vi "Controle_Manip_Main_GUI_WorkingBackup_211222.vi"() -> ()   [LabVIEW 2019] (continued)
                      n490 = property class="Page"(reference=w548, "PageVis"=TRUE ("Page Visible")) -> ()  [unwired: 1 in, 2 out]
                      n491 = property class="Page"(reference=w552, "PageVis"=TRUE ("Page Visible")) -> ()  [unwired: 1 in, 2 out]
                    }
                    frame False {
                      n492 = property on="Experimental parameters tab" class="TabCtl (strict)"() -> ("Pages"=w557:refnum<vi>[])  [unwired: 2 in, 2 out]
                      n493 = property on="Experiment Graph Controls" class="TabCtl (strict)" props=["Value", "Pages"]() -> ("Pages"=w558:refnum<vi>[])  [unwired: 2 in, 3 out]
                      n494 = Index Array(array=w557, index=3) -> (element=w556:refnum<vi>)
                      n495 = Index Array(array=w558, index=3) -> (element=w560:refnum<vi>)
                      n496 = property class="Page"(reference=w556, "PageVis"=FALSE ("Page Visible")) -> ()  [unwired: 1 in, 2 out]
                      n497 = property class="Page"(reference=w560, "PageVis"=FALSE ("Page Visible")) -> ()  [unwired: 1 in, 2 out]
                    }
                  }
                }
                frame True {
                  n498 = stacked-sequence {
                    frame #0 {
                      w577 = TRUE
                      w576 = FALSE
                      n499 = property on="Experiment Graph Controls" class="TabCtl (strict)"("Value"=T25."Contrast" ("Experiment Graph Controls")) -> ("Pages"=w572:refnum<vi>[])  [unwired: 2 in, 2 out]
                      n500 = property on="Experimental parameters tab" class="TabCtl (strict)"("Value"=T19."Translation" ("Experimental parameters tab")) -> ("Pages"=w571:refnum<vi>[])  [unwired: 2 in, 2 out]
                      n501 = local read "Log file"() -> (w567:string)
                      n502 = Index Array(array=w572, index=3) -> (element=w574:refnum<vi>)
                      n503 = Index Array(array=w571, index=3) -> (element=w568:refnum<vi>)
                      n504 = property class="Page"(reference=w574, "PageVis"=TRUE ("Page Visible")) -> ()  [unwired: 1 in, 2 out]
                      n505 = property on="Stop Contrast" class="Bool (strict)"("Visible"=w576) -> ()  [unwired: 2 in, 2 out]
                      n506 = property on="Pause Contrast" class="Bool (strict)"("Visible"=w576) -> ()  [unwired: 2 in, 2 out]
                      n507 = property class="Page"(reference=w568, "PageVis"=TRUE ("Page Visible")) -> ()  [unwired: 1 in, 2 out]
                      n508 = call "Write2LogFile.vi"("Add to log file"="Initialise communication with PZC", "Log file before"=w567, "Checkbox"=FALSE) -> ("Log file after"=w566:string)
                      n509 = local write "Log file"(w566) -> ()
                      n510 = local read "Scan Contrast Ctrls"() -> (w579:refnum<vi>[])
                      n511 = property on="Save Contrast" class="Bool (strict)"("Visible"=w577) -> ()  [unwired: 2 in, 2 out]
                      n512 = property on="Acquire Contrast" class="Bool (strict)"("Visible"=w577) -> ()  [unwired: 2 in, 2 out]
                      n513 = call "Enable&Disable_Controls.vi"("Enum"=enum16{"Enabled", "Disabled", "Disabled&Grayed"}."Enabled", "References"=w579) -> ()  [unwired: 1 in]
                    }
                    frame #1 {
                      # "RS232/10"
                      n514 = local read "PZC200 COM Port"() -> (w581:dbl)
                      n515 = call "Create Instrument Channel.vi"("XON/XOFF Handshaking(F)"=TRUE, "Baud Rate (38400)"=u32 19200, "COM Port (1)"=w581, "(T) - GPIB, F - RS232"=FALSE) -> ("Instrument Channel out"=w585:string)  [unwired: 5 in, 2 out]
                      n516 = call "SendCommand.vi"("Command"="1TS?", "Instrument Channel"=w585) -> ("Instrument Channel out"=w586:string)  [unwired: 8 in, 1 out]
                      n517 = call "ReadCommand.vi"("Disable MAV check (F)"=TRUE, "Instrument Channel"=w586) -> ("Response"=w587:string, "Instrument Channel out"=w580:string)  [unwired: 7 in, 1 out]
                      "Response" <- w587
                      n518 = String Length(string=w587) -> (length=w594:i32)
                      n519 = Subtract(x=w594, y=1) -> (x-y=w592:i32)
                      n520 = local write "PZC200 Instrument Channel"(w580) -> ()
                      n521 = String Subset(string=w587, offset (0)=w592) -> (substring=w591:string)  [unwired: 1 in]
                      n522 = case shown="\"@\", Default" w591 {
                        tunnel: [FALSE TRUE TRUE] -> w590
                        frame "@", Default {
                        }
                        frame "Q" {
                        }
                        frame "P" {
                        }
                      }
                      n523 = local write "LinTFine Motor On?"(w590) -> ()
                      n524 = call "PZCGetPos.vi"("Instrument Channel"=w580) -> ("Position"=w588:i32)  [unwired: 1 in, 2 out]
                      n525 = local write "PZC Position Readout (usteps)"(w588) -> ()
                    }
                  }
                }
              }
            }
            frame #15 {
              # "Advance progress bar"
              n526 = local write "Scan Main Progess Bar"(u8 85 ("Scan Main Progess Bar")) -> ()
            }
            frame #16 {
              # "Attocube ANC350 with 2 ANPx51 and 1 ANPz51"
              n527 = case shown="True" "Attocubes On?" {
                tunnel: [FALSE ("Page Visible") TRUE] -> w600
                frame False {
                }
                frame True {
                  n528 = stacked-sequence {
                    frame #0 {
                      n529 = control-ref of="Experimental parameters tab"() -> (w610:refnum<vi>)
                      n530 = property class="TabCtl (strict)"(reference=w610, "Value"=T19."Microscope objective") -> ()  [unwired: 1 in, 2 out]
                      n531 = local read "Log file"() -> (w614:string)
                      n532 = control-ref of="Tab Objective Sample"() -> (w612:refnum<vi>)
                      n533 = call "Write2LogFile.vi"("Add to log file"="Initialise communication with ANC350", "Log file before"=w614, "Checkbox"=FALSE) -> ("Log file after"=w615:string)
                      n534 = local write "Log file"(w615) -> ()
                      n535 = property class="TabCtl (strict)"(reference=w612, "Value"=T22."Sample piezo stack") -> ()  [unwired: 1 in, 2 out]
                      "ourDLL" <- path "C:/Users/manip/Documents/Controle_Manip_2020/subVIs/Attocubes/anc350v4.dll"
                    }
                    frame #1 {
                      w620 = u32 1 items=["None", "USB", "TCP", "All"] ("Interface types")
                      n536 = local read "ourDLL"() -> (w617:path)
                      n537 = call "ANC350v4_Discover.vi"("Path to *.DLL"=w617, "Interface types"=w620) -> ("ANC350v4 found"=w619:u32, "error ANC350v4_discover"=w618:errorcluster)  [unwired: 12 in]
                      n538 = case shown="1" w619 {
                        tunnel: w618 -> [_ w622]
                        tunnel: w617 -> [_ w621]
                        frame 0, Default {
                        }
                        frame 1 {
                          n539 = stacked-sequence {
                            seq-local: [w624 _] -> [_ w655]
                            seq-local: [w623 _] -> [_ w654]
                            tunnel: w622 -> [w641 _]
                            tunnel: w621 -> [w630 w653]
                            frame #0 {
                              w625 = u8 0 items=["1", "2", "3"] ("axis")
                              w628 = u8 2 items=["1", "2", "3"] ("axis")
                              w629 = u8 1 items=["1", "2", "3"] ("axis")
                              n540 = call "ANC350v4sub_Connect.vi"("Path to *.DLL"=w630, "deviceNumber"=0, "error in"=w641) -> ("ANC350v4_Handle_Out"=w637:u64, "error ANC350v4_Dis/Connect"=w640:errorcluster)  [unwired: 11 in]
                              n541 = call "ANC350v4_GetDeviceInfo.vi"("Path to *.DLL"=w630, "deviceNumber"=u32 0, "error in"=w640) -> ("connected"=→"ANC connected":bool, "Error_ANC350v4_getDeviceInfo"=w636:errorcluster)  [unwired: 5 in, 6 out]
                              n542 = call "ANC350v4_GetPosition.vi"("deviceHandle"=w637, "Path to *.DLL"=w630, "axis"=w625, "error in"=w636) -> ("deviceHandle"=w634:u64, "Position [µm | m°]"=w635:dbl, "error ANC350v4_getPosition"=w633:errorcluster)  [unwired: 8 in, 1 out]
                              n543 = local write "Att Pos Y"(w635) -> ()
                              n544 = call "ANC350v4_GetPosition.vi"("deviceHandle"=w634, "Path to *.DLL"=w630, "axis"=w629, "error in"=w633) -> ("deviceHandle"=w632:u64, "Position [µm | m°]"=w626:dbl, "error ANC350v4_getPosition"=w631:errorcluster)  [unwired: 8 in, 1 out]
                              n545 = local write "Att Pos X"(w626) -> ()
                              n546 = call "ANC350v4_GetPosition.vi"("deviceHandle"=w632, "Path to *.DLL"=w630, "axis"=w628, "error in"=w631) -> ("deviceHandle"=w624:u64, "Position [µm | m°]"=w627:dbl, "error ANC350v4_getPosition"=w623:errorcluster)  [unwired: 8 in, 1 out]
                              n547 = local write "Att Pos Z"(w627) -> ()
                            }
                            frame #1 {
                              w643 = u8 2 items=["1", "2", "3"] ("axis")
                              w644 = u8 1 items=["1", "2", "3"] ("axis")
                              w645 = u8 0 items=["1", "2", "3"] ("axis")
                              w652 = 0.1 ("TargetRange [µm | m°]")
                              # "Define Target resolution in um"
                              n548 = call "ANC350v4_SetTargetRange.vi"("deviceHandle"=w655, "Path to *.DLL"=w653, "axis"=w645, "TargetRange [µm | m°]"=w652, "error in"=w654) -> ("deviceHandle"=w651:u64, "error ANC350v4_setTargetRange"=w649:errorcluster)  [unwired: 8 in, 1 out]
                              n549 = call "ANC350v4_SetTargetRange.vi"("deviceHandle"=w651, "Path to *.DLL"=w653, "axis"=w644, "TargetRange [µm | m°]"=w652, "error in"=w649) -> ("deviceHandle"=w650:u64, "error ANC350v4_setTargetRange"=w648:errorcluster)  [unwired: 8 in, 1 out]
                              n550 = call "ANC350v4_SetTargetRange.vi"("deviceHandle"=w650, "Path to *.DLL"=w653, "axis"=w643, "TargetRange [µm | m°]"=w652, "error in"=w648) -> ("deviceHandle"=→"Att DeviceHandle":u64, "error ANC350v4_setTargetRange"=→"Att Error":errorcluster)  [unwired: 8 in, 1 out]
                            }
                          }
                        }
                      }
                    }
                  }
                }
              }
              n551 = control-ref of="Tab Objective Sample"() -> (w602:refnum<vi>)
              n552 = property class="TabCtl (strict)"(reference=w602) -> ("Pages"=w603:refnum<vi>[])  [unwired: 1 in, 2 out]
              n553 = Index Array(array=w603, index=1) -> (element=w604:refnum<vi>)
              n554 = property class="Page"(reference=w604, "PageVis"=w600) -> ()  [unwired: 1 in, 2 out]
            }
            frame #17 {
              # "Montana Cryostation s50"
              n555 = case shown="True" "Cryostation On?" {
                frame False {
                }
                frame True {
                  w671 = 10.0 ("y")
                  n556 = call "CryoConnect.vi"() -> ("connection ID"=w661:refnum<k5>)
                  "Cryostation ID" <- w661
                  n557 = local read "Log file"() -> (w660:string)
                  n558 = call "Write2LogFile.vi"("Add to log file"="Initialise communication with Cryostation", "Log file before"=w660, "Checkbox"=FALSE) -> ("Log file after"=w659:string)
                  n559 = local write "Log file"(w659) -> ()
                  n560 = call "GetCryoInfo.vi"("connection ID"=w661) -> ("User Stability"=w666:dbl, "User Temp"=w665:dbl, "connection ID out"=w667:refnum<k5>, "Sample Stability"=w664:dbl, "Sample Temp"=w668:dbl, "Platform Stability"=w663:dbl, "Platform Temp"=w662:dbl)  [unwired: 4 in]
                  n561 = local write "Cryo Platform Temp"(w662) -> ()
                  n562 = Multiply(x=w668, y=w671) -> (x*y=w669:dbl)
                  n563 = local write "Cryo Sample Stability"(w664) -> ()
                  n564 = local write "Cryostation ID"(w667) -> ()
                  n565 = local write "Cryo User Stability"(w666) -> ()
                  n566 = local write "Cryo Sample Temp"(w668) -> ()
                  n567 = local write "Cryo Platform Stability"(w663) -> ()
                  n568 = local write "Cryo User Temp"(w665) -> ()
                  n569 = Round To Nearest(number=w669) -> (nearest integer value=w670:dbl)
                  n570 = Divide(x=w670, y=w671) -> (x/y=w672:dbl)
                  n571 = local write "Temperature (K)"(w672) -> ()
                }
              }
            }
            frame #18 {
              # "PicoHarp"
              n572 = case shown="True" "PicoHarp On?" {
                frame False {
                  n573 = local write "Connected"(FALSE) -> ()
                }
                frame True {
                  n574 = local read "Log file"() -> (w684:string)
                  n575 = property on="Experiment Graph Controls" class="TabCtl (strict)"("Value"=T25."APDs" ("Experiment Graph Controls")) -> ("Pages"=w679:refnum<vi>[])  [unwired: 2 in, 2 out]
                  n576 = call "Write2LogFile.vi"("Add to log file"="Initialise communication with PicoHarp", "Log file before"=w684, "Checkbox"=FALSE) -> ("Log file after"=w683:string)
                  n577 = call "PH_Init.vi"() -> ("PH_Init_Data"=→"PH_Init_Data":T11)
                  n578 = local write "Log file"(w683) -> ()
                  n579 = Index Array(array=w679, index=4) -> (element=w680:refnum<vi>)
                  n580 = property class="Page"(reference=w680, "PageVis"=TRUE ("Page Visible")) -> ()  [unwired: 1 in, 2 out]
                  n581 = local write "Connected"(TRUE) -> ()
                }
              }
            }
            frame #19 {
              # "Final activation message"
              n582 = local read "Log file"() -> (w690:string)
              n583 = property on="Experiment Graph Controls" class="TabCtl (strict)"("Value"=T25."Settings" ("Experiment Graph Controls")) -> ()  [unwired: 2 in, 2 out]
              n584 = call "Write2LogFile.vi"("Add to log file"="All devices activated !", "Log file before"=w690, "Checkbox"=FALSE) -> ("Log file after"=w691:string)
              n585 = local write "Log file"(w691) -> ()
              n586 = local write "Scan Main Progess Bar"(u8 100 ("Scan Main Progess Bar")) -> ()
            }
            frame #20 {
              # "Autosave Init"
              n587 = local read "Auto< ?"() -> (w692:bool)
              n588 = case shown="True" w692 {
                frame False {
                  w693 = TRUE ("Visible")
                  n589 = property on="Save Spectrum N" class="Bool (strict)"("Visible"=w693) -> ()  [unwired: 2 in, 2 out]
                  n590 = property on="Save XY Map" class="Bool (strict)"("Visible"=w693) -> ()  [unwired: 2 in, 2 out]
                  n591 = property on="Save Spectrum" class="Bool (strict)"("Visible"=w693) -> ()  [unwired: 2 in, 2 out]
                  n592 = property on="Save PLE" class="Bool (strict)"("Visible"=w693) -> ()  [unwired: 2 in, 2 out]
                  n593 = property on="Save fPow" class="Bool (strict)"("Visible"=w693) -> ()  [unwired: 2 in, 2 out]
                  n594 = property on="Save Custom Diode Spectrum" class="Bool (strict)"("Visible"=w693) -> ()  [unwired: 2 in, 2 out]
                  n595 = property on="Save Michelson" class="Bool (strict)"("Visible"=w693) -> ()  [unwired: 2 in, 2 out]
                  n596 = property on="Save Polarisation" class="Bool (strict)"("Visible"=w693) -> ()  [unwired: 2 in, 2 out]
                  n597 = property on="Save Contrast" class="Bool (strict)"("Visible"=w693) -> ()  [unwired: 2 in, 2 out]
                }
                frame True {
                  w694 = FALSE ("Visible")
                  n598 = property on="Save Spectrum N" class="Bool (strict)"("Visible"=w694) -> ()  [unwired: 2 in, 2 out]
                  n599 = property on="Save XY Map" class="Bool (strict)"("Visible"=w694) -> ()  [unwired: 2 in, 2 out]
                  n600 = property on="Save Spectrum" class="Bool (strict)"("Visible"=w694) -> ()  [unwired: 2 in, 2 out]
                  n601 = property on="Save PLE" class="Bool (strict)"("Visible"=w694) -> ()  [unwired: 2 in, 2 out]
                  n602 = property on="Save fPow" class="Bool (strict)"("Visible"=w694) -> ()  [unwired: 2 in, 2 out]
                  n603 = property on="Save Polarisation" class="Bool (strict)"("Visible"=w694) -> ()  [unwired: 2 in, 2 out]
                  n604 = property on="Save Michelson" class="Bool (strict)"("Visible"=w694) -> ()  [unwired: 2 in, 2 out]
                  n605 = property on="Save Contrast" class="Bool (strict)"("Visible"=w694) -> ()  [unwired: 2 in, 2 out]
                  n606 = property on="Save Custom Diode Spectrum" class="Bool (strict)"("Visible"=w694) -> ()  [unwired: 2 in, 2 out]
                }
              }
            }
          }
        }
      }
    }
    frame #2 {
      # "Main Program"
      n607 = while {
        stop <- w846 stop-if-true
        # "Main loop with unique event structure handling nearly all events (that needn't happen at the same time)"
        n608 = event shown="[0] \"Acquire Time Trace\", \"Acquire Polarisation\", \"Acquire XY Map\", \"Acquire Contrast\", \"Acquire Michelson\", \"Acquire Spectrum\", \"Fast Acq\", \"Acquire Custom Diode Spectrum\", \"Acquire fPow\", \"Acquire PLE\": Mouse Down" {
          selector: _ -> [_ _ _ _ _ _ _ _ _ _ _ _ _ _ _ _ _ _ _ _ _ _ _ _ _ _ _ _ _ _ _ _ _ _ _ _ _ _ _ _ _ _ _ _ _ _ _ _ _ _ _ _ _ _]
          dyn-events: _ -> [_ _ _ _ _ _ _ _ _ _ _ _ _ _ _ _ _ _ _ _ _ _ _ _ _ _ _ _ _ _ _ _ _ _ _ _ _ _ _ _ _ _ _ _ _ _ _ _ _ _ _ _ _ _]
          timeout: 500 -> [_ _ _ _ _ _ _ _ _ _ _ _ _ _ _ _ _ _ _ _ _ _ _ _ _ _ _ _ _ _ _ _ _ _ _ _ _ _ _ _ _ _ _ _ _ _ _ _ _ _ _ _ _ _]
          tunnel: [_ _ _ _ _ _ _ _ _ _ _ _ _ _ _ _ _ _ _ _ _ _ _ _ _ _ _ _ _ _ _ _ _ _ _ _ _ _ _ _ _ _ _ _ _ _ _ _ w4459 _ _ _ _ _] -> w846
          event "Acquire Time Trace", "Acquire Polarisation", "Acquire XY Map", "Acquire Contrast", "Acquire Michelson", "Acquire Spectrum", "Fast Acq", "Acquire Custom Diode Spectrum", "Acquire fPow", "Acquire PLE": Mouse Down {
            # "FAILLE\naucune protection \nde trigger si ESP et \nPicoHarp mais pas LF"
            # "Launch an acquisition or an experiment"
            n609 = event-data() -> ("CtlRef"=w852:refnum<vi>)  [unwired: 1 in, 7 out]
            n610 = local read "LightField On?"() -> (w849:bool)
            n611 = local read "PicoHarp On?"() -> (w850:bool)
            n612 = local read "ESP 300 On?"() -> (w851:bool)
            n613 = And(x=w851, y=w850) -> (x .and. y?=w848:bool)
            n614 = Or(x=w849, y=w848) -> (x .or. y?=w847:bool)
            n615 = stacked-sequence {
              tunnel: w852 -> [w854 w2750]
              tunnel: w847 -> [w853 _]
              frame #0 {
                # "Actual measurements"
                n616 = case shown="True" w853 {
                  tunnel: w854 -> [_ w859]
                  frame False {
                    n617 = local read "Log file"() -> (w858:string)
                    n618 = call "Write2LogFile.vi"("Add to log file"="LightField not activated; cannot acquire", "Log file before"=w858, "Checkbox"=FALSE) -> ("Log file after"=w857:string)
                    n619 = local write "Log file"(w857) -> ()
                  }
                  frame True {
                    n620 = property class="Bool"(reference=w859) -> ("Label.Text"=w860:string)  [unwired: 1 in, 2 out]
                    n621 = case shown="\"Acquire XY Map\"" w860 {
                      frame "Acquire Spectrum", Default {
                        n622 = stacked-sequence {
                          frame #0 {
                            # "background"
                            n623 = local read "Background taken?"() -> (w861:bool)
                            n624 = case shown="False" w861 {
                              frame False {
                                n625 = stacked-sequence {
                                tunnel: [_ _ w907] -> w862
                                frame #0 {
                                n626 = property on="CCD 1D Spectrum Main" class="XYGraph (strict)"("YScale.Offset"=0.0 ("Y Scale.Offset and Multiplier:Offset")) -> ()  [unwired: 2 in, 2 out]
                                }
                                frame #1 {
                                # "make sure shutter is closed"
                                n627 = local read "KCube Shutter On?"() -> (w893:bool)
                                n628 = control-ref of="Shutter Ctrls"() -> (w897:refnum<vi>)
                                n629 = property class="Ring (strict)"(reference=w897) -> ("Value"=w896:u16)  [unwired: 1 in, 2 out]
                                n630 = control-ref of="KCube Shutter Device Reference"() -> (w898:refnum<vi>)
                                n631 = Equal?(x=w896, y=u16 0) -> (x = y?=w894:bool)
                                n632 = case shown="False" w894 {
                                tunnel: w898 -> [w901 _]
                                tunnel: w897 -> [w900 _]
                                tunnel: w893 -> [w899 _]
                                frame False {
                                n633 = call "Shutter.vi"("KCube Shutter Device Reference 2"=w901, "Shutter Ctrls 2"=w900, "Shutter on?"=w899) -> ()
                                }
                                frame True {
                                }
                                }
                                }
                                frame #2 {
                                # "acquire"
                                n634 = local read "LightField Automation error out"() -> (w905:errorcluster)
                                n635 = local read "LightField Automation out"() -> (w906:refnum<class "LightField Automation.lvclass">)
                                n636 = local read "Accumulations"() -> (w902:dbl)
                                n637 = call "LFA_Capture.vi"("error in (no error)"=w905, "Frames"=w902, "LightField Automation in"=w906) -> ("error out"=w904:errorcluster, "Data"=w907:T26, "LightField Automation out"=w903:refnum<class "LightField Automation.lvclass">)  [unwired: 6 in]
                                n638 = local write "LightField Automation error out"(w904) -> ()
                                n639 = local write "LightField Automation out"(w903) -> ()
                                }
                                }
                                n640 = local read "Acq Mode"() -> (w863:T3)
                                n641 = case shown="\"Spectrum\", Default" w863 {
                                selector: w863 -> [w864 w882]
                                tunnel: w862 -> [w865 w883]
                                frame "Spectrum", Default {
                                n642 = stacked-sequence {
                                tunnel: w865 -> [_ w876 _ _]
                                tunnel: w864 -> [_ w874 _ _]
                                frame #0 {
                                n643 = property on="CCD 2D Image Main" class="IntGraph (strict)"("Visible"=FALSE) -> ()  [unwired: 2 in, 2 out]
                                n644 = property on="CCD 1D Spectrum Main" class="XYGraph (strict)"("Visible"=TRUE) -> ()  [unwired: 2 in, 2 out]
                                }
                                frame #1 {
                                n645 = local read "Wavelength calibration"() -> (w873:dbl[])
                                n646 = local read "CCD ROI"() -> (w869:T20)
                                n647 = Divide(x=1239.842, y=w873) -> (x/y=w871:dbl[])
                                n648 = call "PrepareData4Graph.vi"("Wavelength nm"=w871, "DataLF"=w876, "CCD ROI"=w869, "AcqMode"=w874, "Data type"=T30."Spectre") -> ("Spectrum"=w875:cluster{"Array 2":dbl[], "Array":dbl[]}, "PLInt out"=w868:dbl[])  [unwired: 2 in, 2 out]
                                n649 = local write "CCD 1D Spectrum Main"(w875) -> ()
                                n650 = local write "BackgroundSpec"(w868) -> ()
                                }
                                frame #2 {
                                n651 = local read "BackgroundSpec"() -> (w877:dbl[])
                                n652 = call-poly <vilib>:"Mean.vi"("X"=w877) -> ("mean"=w879:dbl)  [unwired: 1 out]
                                n653 = Negate(x=w879) -> (-x=w878:dbl)
                                n654 = property on="CCD 1D Spectrum Main" class="XYGraph (strict)"("YScale.Offset"=w878) -> ()  [unwired: 2 in, 2 out]
                                }
                                frame #3 {
                                n655 = local write "Background taken?"(TRUE ("Background taken?")) -> ()
                                n656 = property on="Background substract" class="Enum (strict)"("Value"=enum16{"None", "Shutter"}."None" ("Background substract")) -> ()  [unwired: 2 in, 2 out]
                                }
                                }
                                }
                                frame "Image" {
                                n657 = stacked-sequence {
                                tunnel: w883 -> [_ w891]
                                tunnel: w882 -> [_ w889]
                                frame #0 {
                                n658 = property on="CCD 1D Spectrum Main" class="XYGraph (strict)"("Visible"=FALSE) -> ()  [unwired: 2 in, 2 out]
                                n659 = property on="CCD 2D Image Main" class="IntGraph (strict)"("Visible"=TRUE) -> ()  [unwired: 2 in, 2 out]
                                }
                                frame #1 {
                                n660 = local read "Wavelength calibration"() -> (w890:dbl[])
                                n661 = local read "CCD ROI"() -> (w886:T20)
                                n662 = call "PrepareData4Graph.vi"("Wavelength nm"=w890, "DataLF"=w891, "CCD ROI"=w886, "AcqMode"=w889, "Data type"=T30."Spectre") -> ("Intensity Graph"=w888:dbl[][])  [unwired: 2 in, 3 out]
                                n663 = local write "CCD 2D Image Main"(w888) -> ()
                                }
                                }
                                }
                                }
                              }
                              frame True {
                              }
                            }
                          }
                          frame #1 {
                            # "measurement"
                            n664 = stacked-sequence {
                              frame #0 {
                                # "open shutter if closed"
                                n665 = control-ref of="KCube Shutter Device Reference"() -> (w910:refnum<vi>)
                                n666 = control-ref of="Shutter Ctrls"() -> (w909:refnum<vi>)
                                n667 = property class="Ring (strict)"(reference=w909) -> ("Value"=w911:u16)  [unwired: 1 in, 2 out]
                                n668 = local read "KCube Shutter On?"() -> (w914:bool)
                                n669 = Equal?(x=w911, y=u16 0) -> (x = y?=w913:bool)
                                n670 = property on="Experiment Graph Controls" class="TabCtl (strict)"("Value"=T25."Spectrum" ("Experiment Graph Controls")) -> ()  [unwired: 2 in, 2 out]
                                n671 = case shown="True" w913 {
                                tunnel: w910 -> [_ w917]
                                tunnel: w909 -> [_ w916]
                                tunnel: w914 -> [_ w915]
                                frame False {
                                }
                                frame True {
                                n672 = call "Shutter.vi"("KCube Shutter Device Reference 2"=w917, "Shutter Ctrls 2"=w916, "Shutter on?"=w915) -> ()
                                }
                                }
                              }
                              frame #1 {
                                # "set CCD ROI and acquire"
                                n673 = local read "LightField Automation error out"() -> (w926:errorcluster)
                                n674 = local read "LightField Automation out"() -> (w918:refnum<class "LightField Automation.lvclass">)
                                n675 = local read "CCD ROI"() -> (w925:T20)
                                n676 = local read "Accumulations"() -> (w922:dbl)
                                n677 = call "Adv_SetROI.vi"("error in (no error)"=w926, "ROI"=w925, "LightField Automation in"=w918) -> ("error out"=w923:errorcluster, "LightField Automation out"=w924:refnum<class "LightField Automation.lvclass">)  [unwired: 7 in]
                                n678 = call "LFA_Capture.vi"("error in (no error)"=w923, "Frames"=w922, "LightField Automation in"=w924) -> ("error out"=w921:errorcluster, "Data"=w920:T26, "LightField Automation out"=w919:refnum<class "LightField Automation.lvclass">)  [unwired: 6 in]
                                n679 = local write "LightField Automation out"(w919) -> ()
                                n680 = local write "LightField Automation error out"(w921) -> ()
                                n681 = local write "Data"(w920) -> ()
                              }
                              frame #2 {
                                # "close shutter"
                                n682 = local read "KCube Shutter On?"() -> (w929:bool)
                                n683 = control-ref of="KCube Shutter Device Reference"() -> (w928:refnum<vi>)
                                n684 = control-ref of="Shutter Ctrls"() -> (w927:refnum<vi>)
                                n685 = call "Shutter.vi"("KCube Shutter Device Reference 2"=w928, "Shutter Ctrls 2"=w927, "Shutter on?"=w929) -> ()
                              }
                              frame #3 {
                                # "Show data accordingly"
                                n686 = local read "Data"() -> (w930:T26)
                                n687 = local read "Acq Mode"() -> (w931:T3)
                                n688 = case shown="\"Spectrum\", Default" w931 {
                                selector: w931 -> [w932 w951]
                                tunnel: w930 -> [w933 w952]
                                frame "Spectrum", Default {
                                n689 = stacked-sequence {
                                tunnel: w933 -> [_ w949 _]
                                tunnel: w932 -> [_ w948 _]
                                frame #0 {
                                n690 = property on="CCD 1D Spectrum Main" class="XYGraph (strict)"("Visible"=TRUE) -> ()  [unwired: 2 in, 2 out]
                                n691 = property on="CCD 2D Image Main" class="IntGraph (strict)"("Visible"=FALSE) -> ()  [unwired: 2 in, 2 out]
                                }
                                frame #1 {
                                n692 = local read "Wavelength calibration"() -> (w947:dbl[])
                                n693 = local read "CCD ROI"() -> (w943:T20)
                                n694 = local read "BackgroundSpec"() -> (w937:dbl[])
                                n695 = Divide(x=1239.842, y=w947) -> (x/y=w945:dbl[])
                                n696 = call "PrepareData4Graph.vi"("BackgroundSpec"=w937, "Wavelength nm"=w945, "DataLF"=w949, "CCD ROI"=w943, "AcqMode"=w948, "Data type"=T30."Spectre") -> ("Spectrum"=w936:cluster{"Array 2":dbl[], "Array":dbl[]}, "PLInt out"=w941:dbl[])  [unwired: 1 in, 2 out]
                                n697 = control-ref of="Cnts"() -> (w942:refnum<vi>)
                                n698 = local read "Excitation Power (uW)"() -> (w939:dbl)
                                n699 = local write "CCD 1D Spectrum Main"(w936) -> ()
                                n700 = local read "Acq Time (ms)"() -> (w940:dbl)
                                n701 = local read "Display Mode"() -> (w938:u16)
                                n702 = call "2Cnts.vi"("Array Background"=w937, "Pow W"=w939, "AcqTime ms"=w940, "Cnts Ref"=w942, "Display Mode"=w938, "Array"=w941) -> ()  [unwired: 1 out]
                                }
                                frame #2 {
                                n703 = property on="Full scale" class="Bool (strict)"("Val(Sgnl)"=TRUE ("Value (Signaling)")) -> ()  [unwired: 2 in, 2 out]
                                }
                                }
                                }
                                frame "Image" {
                                n704 = stacked-sequence {
                                tunnel: w952 -> [_ w960]
                                tunnel: w951 -> [_ w958]
                                frame #0 {
                                n705 = property on="CCD 1D Spectrum Main" class="XYGraph (strict)"("Visible"=FALSE) -> ()  [unwired: 2 in, 2 out]
                                n706 = property on="CCD 2D Image Main" class="IntGraph (strict)"("Visible"=TRUE) -> ()  [unwired: 2 in, 2 out]
                                }
                                frame #1 {
                                n707 = local read "Wavelength calibration"() -> (w959:dbl[])
                                n708 = local read "CCD ROI"() -> (w955:T20)
                                n709 = call "PrepareData4Graph.vi"("Wavelength nm"=w959, "DataLF"=w960, "CCD ROI"=w955, "AcqMode"=w958, "Data type"=T30."Spectre") -> ("Intensity Graph"=w957:dbl[][])  [unwired: 2 in, 3 out]
                                n710 = local write "CCD 2D Image Main"(w957) -> ()
                                }
                                }
                                }
                                }
                              }
                            }
                          }
                        }
                      }
                      frame "Acquire fPow" {
                        n711 = stacked-sequence {
                          frame #0 {
                            # "background"
                            n712 = local read "Background taken?"() -> (w961:bool)
                            n713 = case shown="False" w961 {
                              frame False {
                                n714 = stacked-sequence {
                                tunnel: [_ _ w1007] -> w962
                                frame #0 {
                                n715 = property on="CCD 1D Spectrum Main" class="XYGraph (strict)"("YScale.Offset"=0.0 ("Y Scale.Offset and Multiplier:Offset")) -> ()  [unwired: 2 in, 2 out]
                                }
                                frame #1 {
                                # "make sure shutter is closed"
                                n716 = local read "KCube Shutter On?"() -> (w993:bool)
                                n717 = control-ref of="Shutter Ctrls"() -> (w997:refnum<vi>)
                                n718 = property class="Ring (strict)"(reference=w997) -> ("Value"=w996:u16)  [unwired: 1 in, 2 out]
                                n719 = control-ref of="KCube Shutter Device Reference"() -> (w998:refnum<vi>)
                                n720 = Equal?(x=w996, y=u16 0) -> (x = y?=w994:bool)
                                n721 = case shown="False" w994 {
                                tunnel: w998 -> [w1001 _]
                                tunnel: w997 -> [w1000 _]
                                tunnel: w993 -> [w999 _]
                                frame False {
                                n722 = call "Shutter.vi"("KCube Shutter Device Reference 2"=w1001, "Shutter Ctrls 2"=w1000, "Shutter on?"=w999) -> ()
                                }
                                frame True {
                                }
                                }
                                }
                                frame #2 {
                                # "acquire"
                                n723 = local read "LightField Automation error out"() -> (w1005:errorcluster)
                                n724 = local read "LightField Automation out"() -> (w1006:refnum<class "LightField Automation.lvclass">)
                                n725 = local read "Accumulations"() -> (w1002:dbl)
                                n726 = call "LFA_Capture.vi"("error in (no error)"=w1005, "Frames"=w1002, "LightField Automation in"=w1006) -> ("error out"=w1004:errorcluster, "Data"=w1007:T26, "LightField Automation out"=w1003:refnum<class "LightField Automation.lvclass">)  [unwired: 6 in]
                                n727 = local write "LightField Automation error out"(w1004) -> ()
                                n728 = local write "LightField Automation out"(w1003) -> ()
                                }
                                }
                                n729 = local read "Acq Mode"() -> (w963:T3)
                                n730 = case shown="\"Spectrum\", Default" w963 {
                                selector: w963 -> [w964 w982]
                                tunnel: w962 -> [w965 w983]
                                frame "Spectrum", Default {
                                n731 = stacked-sequence {
                                tunnel: w965 -> [_ w976 _ _]
                                tunnel: w964 -> [_ w974 _ _]
                                frame #0 {
                                n732 = property on="CCD 2D Image Main" class="IntGraph (strict)"("Visible"=FALSE) -> ()  [unwired: 2 in, 2 out]
                                n733 = property on="CCD 1D Spectrum Main" class="XYGraph (strict)"("Visible"=TRUE) -> ()  [unwired: 2 in, 2 out]
                                }
                                frame #1 {
                                n734 = local read "Wavelength calibration"() -> (w973:dbl[])
                                n735 = local read "CCD ROI"() -> (w969:T20)
                                n736 = Divide(x=1239.842, y=w973) -> (x/y=w971:dbl[])
                                n737 = call "PrepareData4Graph.vi"("Wavelength nm"=w971, "DataLF"=w976, "CCD ROI"=w969, "AcqMode"=w974, "Data type"=T30."Spectre") -> ("Spectrum"=w975:cluster{"Array 2":dbl[], "Array":dbl[]}, "PLInt out"=w968:dbl[])  [unwired: 2 in, 2 out]
                                n738 = local write "CCD 1D Spectrum Main"(w975) -> ()
                                n739 = local write "BackgroundSpec"(w968) -> ()
                                }
                                frame #2 {
                                n740 = local read "BackgroundSpec"() -> (w977:dbl[])
                                n741 = call-poly <vilib>:"Mean.vi"("X"=w977) -> ("mean"=w979:dbl)  [unwired: 1 out]
                                n742 = Negate(x=w979) -> (-x=w978:dbl)
                                n743 = property on="CCD 1D Spectrum Main" class="XYGraph (strict)"("YScale.Offset"=w978) -> ()  [unwired: 2 in, 2 out]
                                }
                                frame #3 {
                                n744 = local write "Background taken?"(TRUE ("Background taken?")) -> ()
                                n745 = property on="Background substract" class="Enum (strict)"("Value"=enum16{"None", "Shutter"}."None" ("Background substract")) -> ()  [unwired: 2 in, 2 out]
                                }
                                }
                                }
                                frame "Image" {
                                n746 = stacked-sequence {
                                tunnel: w983 -> [_ w991]
                                tunnel: w982 -> [_ w989]
                                frame #0 {
                                n747 = property on="CCD 1D Spectrum Main" class="XYGraph (strict)"("Visible"=FALSE) -> ()  [unwired: 2 in, 2 out]
                                n748 = property on="CCD 2D Image Main" class="IntGraph (strict)"("Visible"=TRUE) -> ()  [unwired: 2 in, 2 out]
                                }
                                frame #1 {
                                n749 = local read "Wavelength calibration"() -> (w990:dbl[])
                                n750 = local read "CCD ROI"() -> (w986:T20)
                                n751 = call "PrepareData4Graph.vi"("Wavelength nm"=w990, "DataLF"=w991, "CCD ROI"=w986, "AcqMode"=w989, "Data type"=T30."Spectre") -> ("Intensity Graph"=w988:dbl[][])  [unwired: 2 in, 3 out]
                                n752 = local write "CCD 2D Image Main"(w988) -> ()
                                }
                                }
                                }
                                }
                              }
                              frame True {
                              }
                            }
                          }
                          frame #1 {
                            w1013 = TRUE ("Visible")
                            w1014 = FALSE ("Visible")
                            # "init"
                            n753 = control-ref of="N Step Power  Diode Current (A)"() -> (w1017:refnum<vi>)
                            n754 = control-ref of="End Power  Diod Current (A)"() -> (w1018:refnum<vi>)
                            n755 = control-ref of="Start Power Diod Current (A)"() -> (w1019:refnum<vi>)
                            n756 = control-ref of="Acquire fPow"() -> (w1023:refnum<vi>)
                            n757 = control-ref of="Save fPow"() -> (w1021:refnum<vi>)
                            n758 = Build Array(w1023, w1021, w1019, w1018, w1017) -> (w1022:refnum<vi>[])
                            n759 = property on="Elapsed (s)" class="DigNum (strict)"("Visible"=TRUE) -> ()  [unwired: 2 in, 2 out]
                            n760 = call "Enable&Disable_Controls.vi"("Enum"=enum16{"Enabled", "Disabled", "Disabled&Grayed"}."Disabled&Grayed", "References"=w1022) -> ()  [unwired: 1 in]
                            n761 = control-ref of="MasterStop"() -> (w1011:refnum<vi>)
                            n762 = control-ref of="MasterPause"() -> (w1012:refnum<vi>)
                            n763 = control-ref of="Acquire fPow"() -> (w1016:refnum<vi>)
                            n764 = control-ref of="Save fPow"() -> (w1015:refnum<vi>)
                            n765 = property class="Bool (strict)"(reference=w1016, "Visible"=w1014) -> ()  [unwired: 1 in, 2 out]
                            n766 = property class="Bool (strict)"(reference=w1015, "Visible"=w1014) -> ()  [unwired: 1 in, 2 out]
                            n767 = property class="Bool (strict)"(reference=w1011, "Visible"=w1013) -> ()  [unwired: 1 in, 2 out]
                            n768 = property class="Bool (strict)"(reference=w1012, "Visible"=w1013) -> ()  [unwired: 1 in, 2 out]
                            n769 = property on="CCD 2D Image Main" class="IntGraph (strict)"("Visible"=FALSE) -> ()  [unwired: 2 in, 2 out]
                            n770 = property on="CCD 1D Spectrum Main" class="XYGraph (strict)"("Visible"=TRUE) -> ()  [unwired: 2 in, 2 out]
                          }
                          frame #2 {
                            # "measurement"
                            n771 = local read "N Step Power  Diode Current (A)"() -> (w1030:i32)
                            n772 = local read "End Power  Diod Current (A)"() -> (w1034:dbl)
                            n773 = Increment(x=w1030) -> (x+1=w1031:i32)
                            n774 = local read "Start Power Diod Current (A)"() -> (w1032:dbl)
                            n775 = Subtract(x=w1034, y=w1032) -> (x-y=w1033:dbl)
                            n776 = Divide(x=w1033, y=w1030) -> (x/y=w1029:dbl)
                            n777 = for {
                              N: w1031 -> [w1041]
                              tunnel: w1032 -> [w1048]
                              tunnel: w1029 -> [w1047]
                              shift-right: [w1045] -> w1025
                              shift-left: i32[][] [] -> [w1044]
                              shift-right: [w1042] -> w1027
                              shift-left: dbl[] [] -> [w1043]
                              i -> [w1037]
                              stop <- w1035 stop-if-true
                              n778 = Multiply(x=w1037, y=w1047) -> (x*y=w1049:dbl)
                              n779 = Add(x=w1048, y=w1049) -> (x+y=w1046:dbl)
                              n780 = Increment(x=w1037) -> (x+1=w1036:i32)
                              n781 = Divide(x=w1036, y=w1041) -> (x/y=w1040:dbl)
                              n782 = Multiply(x=w1040, y=100.0) -> (x*y=w1038:dbl)
                              n783 = stacked-sequence {
                                tunnel: w1046 -> [w1053 _ _ _ _ _]
                                tunnel: w1044 -> [_ _ _ _ w1110 _]
                                tunnel: [_ _ _ _ w1108 _] -> w1045
                                tunnel: w1043 -> [w1052 _ _ _ _ _]
                                tunnel: [w1050 _ _ _ _ _] -> w1042
                                tunnel: w1038 -> [_ _ _ _ _ w1152]
                                frame #0 {
                                # "set power and wait a bit"
                                n784 = local read "Photodiode handle out"() -> (w1056:refnum<visa-resource-name>)
                                n785 = local read "Photodiode error out"() -> (w1057:errorcluster)
                                n786 = local read "Diode Driver Error"() -> (w1055:errorcluster)
                                n787 = local read "DDE"() -> (w1054:refnum<visa-resource-name>)
                                n788 = stacked-sequence {
                                seq-local: [w1066 _ _] -> [_ _ w1085]
                                seq-local: [w1065 _ _] -> [_ _ w1084]
                                tunnel: w1054 -> [w1070 _ _]
                                tunnel: w1055 -> [w1063 _ _]
                                tunnel: [_ _ w1085] -> w1059
                                tunnel: [_ _ w1084] -> w1061
                                tunnel: w1056 -> [_ _ w1083]
                                tunnel: w1057 -> [_ _ w1082]
                                tunnel: [_ _ w1081] -> w1060
                                tunnel: [_ _ w1080] -> w1058
                                tunnel: w1053 -> [w1062 _ _]
                                tunnel: [_ _ w1079] -> w1051
                                frame #0 {
                                n789 = call <instrlib>:"TL4000 Get Laser Diode Current Setpoint.vi"("error in (no error)"=w1063, "instrument handle"=w1070) -> ("error out"=w1067:errorcluster, "Laser Diode Current Setpoint"=w1069:dbl, "instrument handle out"=w1068:refnum<visa-resource-name>)  [unwired: 7 in]
                                n790 = Not Equal?(x=w1062, y=w1069) -> (x != y?=w1064:bool)
                                n791 = case shown="True" w1064 {
                                tunnel: w1068 -> [w1072 w1077]
                                tunnel: w1067 -> [w1071 w1076]
                                tunnel: [w1072 w1075] -> w1066
                                tunnel: [w1071 w1074] -> w1065
                                tunnel: w1062 -> [_ w1073]
                                frame False {
                                }
                                frame True {
                                n792 = call <instrlib>:"TL4000 Set Laser Diode Current Setpoint.vi"("error in (no error)"=w1076, "Laser Diode Current Setpoint (0.0)"=w1073, "instrument handle"=w1077) -> ("error out"=w1074:errorcluster, "instrument handle out"=w1075:refnum<visa-resource-name>)  [unwired: 7 in]
                                }
                                }
                                }
                                frame #1 {
                                n793 = Wait (ms)(milliseconds to wait=u32 500) -> ()  [unwired: 1 out]
                                }
                                frame #2 {
                                n794 = call <instrlib>:"TLPM Measure Power.vi"("error in (no error)"=w1082, "instrument handle"=w1083) -> ("error out"=w1080:errorcluster, "Power"=w1079:dbl, "instrument handle out"=w1081:refnum<visa-resource-name>)  [unwired: 7 in]
                                n795 = local write "Excitation Power (uW)"(w1079) -> ()
                                }
                                }
                                n796 = Insert Into Array(array=w1052, new element=w1051) -> (w1050:dbl[])  [unwired: 1 in]
                                n797 = local write "Diode Driver Error out"(w1061) -> ()
                                n798 = local write "Photodiode handle out"(w1060) -> ()
                                n799 = local write "Photodiode error out"(w1058) -> ()
                                n800 = local write "Diode Driver COM"(w1059) -> ()
                                }
                                frame #1 {
                                # "open shutter if closed"
                                n801 = control-ref of="KCube Shutter Device Reference"() -> (w1088:refnum<vi>)
                                n802 = control-ref of="Shutter Ctrls"() -> (w1087:refnum<vi>)
                                n803 = property class="Ring (strict)"(reference=w1087) -> ("Value"=w1089:u16)  [unwired: 1 in, 2 out]
                                n804 = local read "KCube Shutter On?"() -> (w1092:bool)
                                n805 = Equal?(x=w1089, y=u16 0) -> (x = y?=w1091:bool)
                                n806 = property on="Experiment Graph Controls" class="TabCtl (strict)"("Value"=T25."Spectrum" ("Experiment Graph Controls")) -> ()  [unwired: 2 in, 2 out]
                                n807 = case shown="True" w1091 {
                                tunnel: w1088 -> [_ w1095]
                                tunnel: w1087 -> [_ w1094]
                                tunnel: w1092 -> [_ w1093]
                                frame False {
                                }
                                frame True {
                                n808 = call "Shutter.vi"("KCube Shutter Device Reference 2"=w1095, "Shutter Ctrls 2"=w1094, "Shutter on?"=w1093) -> ()
                                }
                                }
                                }
                                frame #2 {
                                # "set CCD ROI and acquire"
                                n809 = local read "LightField Automation error out"() -> (w1104:errorcluster)
                                n810 = local read "LightField Automation out"() -> (w1096:refnum<class "LightField Automation.lvclass">)
                                n811 = local read "CCD ROI"() -> (w1103:T20)
                                n812 = local read "Accumulations"() -> (w1100:dbl)
                                n813 = call "Adv_SetROI.vi"("error in (no error)"=w1104, "ROI"=w1103, "LightField Automation in"=w1096) -> ("error out"=w1101:errorcluster, "LightField Automation out"=w1102:refnum<class "LightField Automation.lvclass">)  [unwired: 7 in]
                                n814 = call "LFA_Capture.vi"("error in (no error)"=w1101, "Frames"=w1100, "LightField Automation in"=w1102) -> ("error out"=w1099:errorcluster, "Data"=w1098:T26, "LightField Automation out"=w1097:refnum<class "LightField Automation.lvclass">)  [unwired: 6 in]
                                n815 = local write "LightField Automation out"(w1097) -> ()
                                n816 = local write "LightField Automation error out"(w1099) -> ()
                                n817 = local write "Data"(w1098) -> ()
                                }
                                frame #3 {
                                # "close shutter"
                                n818 = local read "KCube Shutter On?"() -> (w1107:bool)
                                n819 = control-ref of="KCube Shutter Device Reference"() -> (w1106:refnum<vi>)
                                n820 = control-ref of="Shutter Ctrls"() -> (w1105:refnum<vi>)
                                n821 = call "Shutter.vi"("KCube Shutter Device Reference 2"=w1106, "Shutter Ctrls 2"=w1105, "Shutter on?"=w1107) -> ()
                                }
                                frame #4 {
                                # "Show data accordingly"
                                n822 = local read "Data"() -> (w1111:T26)
                                n823 = local read "Acq Mode"() -> (w1112:T3)
                                n824 = case shown="\"Spectrum\", Default" w1112 {
                                selector: w1112 -> [w1114 w1136]
                                tunnel: w1111 -> [w1115 w1137]
                                tunnel: [w1113 w1135] -> w1109
                                frame "Spectrum", Default {
                                n825 = stacked-sequence {
                                tunnel: w1115 -> [_ w1131 _]
                                tunnel: w1114 -> [_ w1129 _]
                                tunnel: [_ w1118 _] -> w1113
                                frame #0 {
                                n826 = property on="CCD 1D Spectrum Main" class="XYGraph (strict)"("Visible"=TRUE) -> ()  [unwired: 2 in, 2 out]
                                n827 = property on="CCD 2D Image Main" class="IntGraph (strict)"("Visible"=FALSE) -> ()  [unwired: 2 in, 2 out]
                                }
                                frame #1 {
                                n828 = local read "Wavelength calibration"() -> (w1128:dbl[])
                                n829 = local read "CCD ROI"() -> (w1124:T20)
                                n830 = Divide(x=1239.842, y=w1128) -> (x/y=w1126:dbl[])
                                n831 = call "PrepareData4Graph.vi"("Wavelength nm"=w1126, "DataLF"=w1131, "CCD ROI"=w1124, "AcqMode"=w1129, "Data type"=T30."Spectre") -> ("Spectrum"=w1130:cluster{"Array 2":dbl[], "Array":dbl[]}, "PLInt out"=w1118:dbl[])  [unwired: 2 in, 2 out]
                                n832 = local write "CCD 1D Spectrum Main"(w1130) -> ()
                                n833 = local read "Excitation Power (uW)"() -> (w1120:dbl)
                                n834 = local read "Acq Time (ms)"() -> (w1121:dbl)
                                n835 = local read "BackgroundSpec"() -> (w1119:dbl[])
                                n836 = local read "Display Mode"() -> (w1122:u16)
                                n837 = control-ref of="Cnts"() -> (w1123:refnum<vi>)
                                n838 = call "2Cnts.vi"("Array Background"=w1119, "Pow W"=w1120, "AcqTime ms"=w1121, "Cnts Ref"=w1123, "Display Mode"=w1122, "Array"=w1118) -> ()  [unwired: 1 out]
                                }
                                frame #2 {
                                n839 = property on="CCD 1D Spectrum Main" class="XYGraph (strict)"() -> ("Value"=w1134:cluster{dbl[], dbl[]})  [unwired: 2 in, 2 out]
                                n840 = Unbundle(w1134) -> (w1133:dbl[])  [unwired: 1 out]
                                n841 = call "myMax.vi"("Array"=w1133) -> ("myMax"=w1132:dbl)  [unwired: 1 in]
                                n842 = property on="CCD 1D Spectrum Main" class="XYGraph (strict)"("YScale.Maximum"=w1132) -> ()  [unwired: 2 in, 2 out]
                                }
                                }
                                }
                                frame "Image" {
                                n843 = stacked-sequence {
                                tunnel: w1137 -> [_ w1151]
                                tunnel: w1136 -> [_ w1149]
                                tunnel: [_ w1140] -> w1135
                                frame #0 {
                                n844 = property on="CCD 1D Spectrum Main" class="XYGraph (strict)"("Visible"=FALSE) -> ()  [unwired: 2 in, 2 out]
                                n845 = property on="CCD 2D Image Main" class="IntGraph (strict)"("Visible"=TRUE) -> ()  [unwired: 2 in, 2 out]
                                }
                                frame #1 {
                                n846 = local read "Wavelength calibration"() -> (w1150:dbl[])
                                n847 = local read "CCD ROI"() -> (w1146:T20)
                                n848 = call "PrepareData4Graph.vi"("Wavelength nm"=w1150, "DataLF"=w1151, "CCD ROI"=w1146, "AcqMode"=w1149, "Data type"=T30."Spectre") -> ("Intensity Graph"=w1148:dbl[][], "PLInt out"=w1140:dbl[])  [unwired: 2 in, 2 out]
                                n849 = local write "CCD 2D Image Main"(w1148) -> ()
                                n850 = local read "Excitation Power (uW)"() -> (w1142:dbl)
                                n851 = local read "Acq Time (ms)"() -> (w1143:dbl)
                                n852 = local read "BackgroundSpec"() -> (w1141:dbl[])
                                n853 = local read "Display Mode"() -> (w1144:u16)
                                n854 = control-ref of="Cnts"() -> (w1145:refnum<vi>)
                                n855 = call "2Cnts.vi"("Array Background"=w1141, "Pow W"=w1142, "AcqTime ms"=w1143, "Cnts Ref"=w1145, "Display Mode"=w1144, "Array"=w1140) -> ()  [unwired: 1 out]
                                }
                                }
                                }
                                }
                                n856 = Insert Into Array(array=w1110, new element=w1109) -> (w1108:i32[][])  [unwired: 2 in]
                                }
                                frame #5 {
                                n857 = local write "Scan Main Progess Bar"(w1152) -> ()
                                n858 = while {
                                stop <- w1153 continue-if-true
                                n859 = Wait (ms)(milliseconds to wait=u32 50) -> ()  [unwired: 1 out]
                                n860 = local read "MasterPause"() -> (w1153:bool)
                                }
                                }
                              }
                              n861 = local read "MasterStop"() -> (w1035:bool)
                            }
                            "Array fPow" <- w1025
                            "Array fPow Pow" <- w1027
                            n862 = Transpose 2D Array(2D array=w1025) -> (transposed array=w1024:i32[][])
                            n863 = property on="CCD 2D Image Main" class="IntGraph (strict)"("Value"=w1024) -> ()  [unwired: 2 in, 2 out]
                          }
                          frame #3 {
                            # "end"
                            n864 = control-ref of="Acquire fPow"() -> (w1167:refnum<vi>)